vi "Interpolate Real.vi"(0 "Bc":dbl=330.0 format="%_4g", 1 "y":dbl=175.0 format="%_4g", 2 "Mag":dbl=50.0 format="%_4g", 3 "theta":ext=1.950013999999992 format="%_4g", 4 "Initial":dbl[](array[numeric])=[535.0, 450.0] format="%_3g", 5 "g0":dbl=0.30979 format="%_3g", 8 "width":dbl=0.04216999999999992 format="%_3g") -> (7 "sum":dbl(knob)=1360414.7194911004 scale=0.0..30000.0)   [LabVIEW 2016]
panel:
  in  "Tab Control":T1(tab)=enum."Data+Fit"
  out "Skeleton":cluster{"B+i Vsg":cdb[]}[](array[cluster])=[{"B+i Vsg"=[535.0+0.0i, 184.2548459187753+306.77613669047014i, 165.7451540812247+353.22386330952986i, -76.67944631491423+535.0i]}, {"B+i Vsg"=[450.0+0.0i, 184.2548459187753+306.77613669047014i, 165.7451540812247+353.22386330952986i, -13.444317955229593+535.0i]}] {"B+i Vsg" format="%_3g"}
  in  "w":dbl[](array[numeric])=[1.0, 1.0, 1.0]
  out "B":dbl=-0.0009832390037923806 format="%_3g"
  out "gcalc":dbl=1.4433966272486396
  out "XY Graph":cluster{dbl[], dbl[]}[](graph)=[{[0.0, 306.77613669047014, 353.22386330952986, 535.0], [535.0, 184.2548459187753, 165.7451540812247, -76.67944631491423]}, {[0.0, 306.77613669047014, 353.22386330952986, 535.0], [450.0, 184.2548459187753, 165.7451540812247, -13.444317955229593]}]
  in  "i final":dbl=535.0
  in  "i initial":dbl
  in  "Bscale":dbl=-1.0
  out "Data - Fit":dbl[][](graph)
  in  "Mask?":bool=TRUE
  out "Fit":dbl[][](graph)
  in  "Data":dbl[][](graph)=array535x467[249845 elements]
  out "Data - Fit Crop":dbl[][](graph)
  in  "Ny":i32=467
  in  "y0":i32
  in  "Nx":i32=535
  in  "x0":i32
  in  "Mask":dbl[][](graph)=array535x467[249845 elements]
  out "Re Out":dbl[](array[numeric])=[-0.05, 0.05, 0.3]
  out "Out":cdb[](array[numeric])=[-0.05+0.0i, 0.05+0.0i, 0.3+0.0i]
  out "size(s) 2":i32[](array[numeric])=[535, 467]
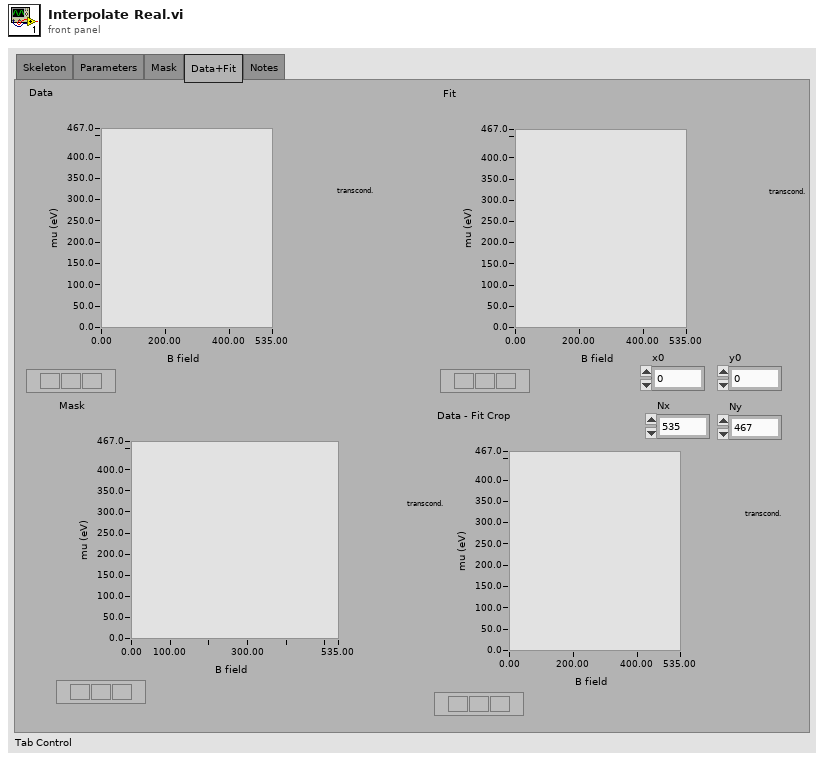
[diagram p1: front panel]
types:
  T1 = enum32{"Skeleton", "Parameters", "Mask", "Data+Fit", "Notes"}
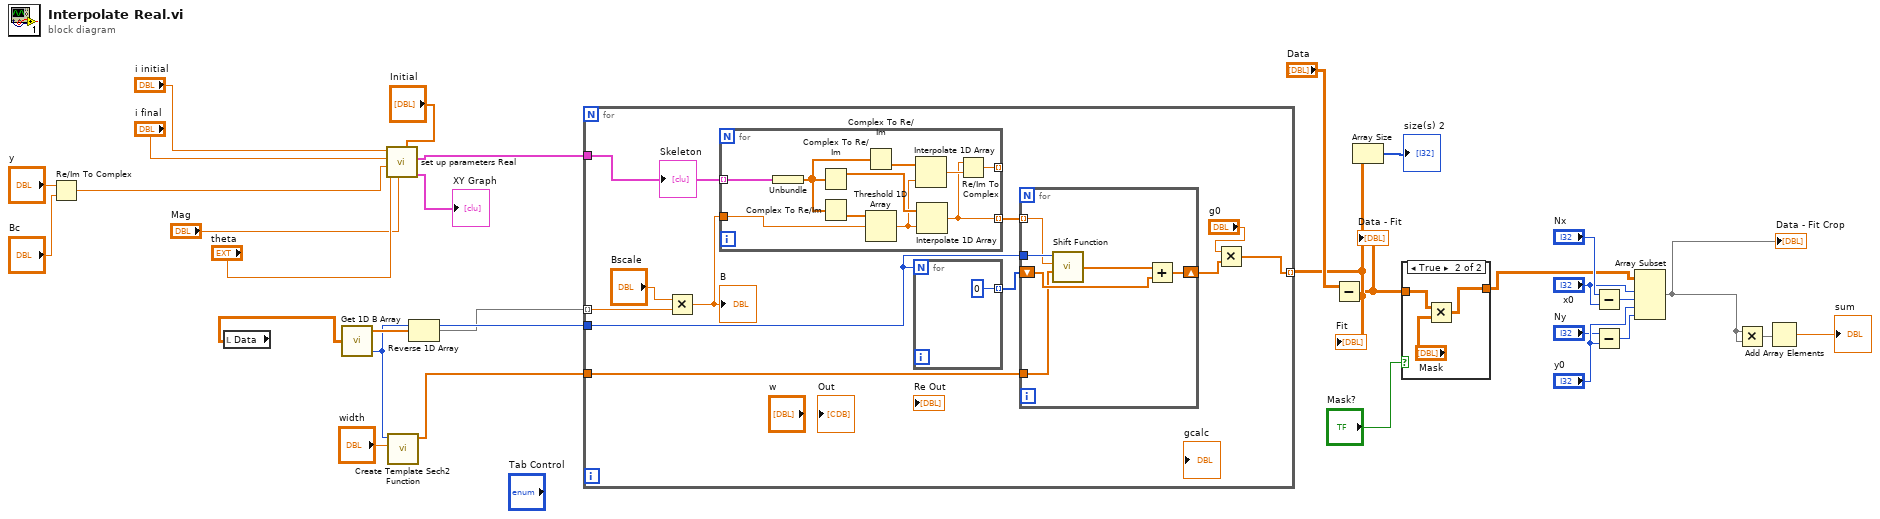
[diagram p0: block diagram]
diagram:
  n1 = Re/Im To Complex(1:"Bc", 2:"y") -> (0:w14:cdb)
  n2 = local read "Data"() -> (w1:dbl[][])
  n3 = call "Get 1D B Array.vi"("B"=w1) -> ("B 1D"=w26:dbl[], "Ny"=w25:i32)  [unwired: 1 out]
  n4 = call "set up parameters Real.vi"("i initial"="i initial", "i final"="i final", "X-point"=w14, "theta"="theta", "Mag"="Mag", "Initial"="Initial") -> ("Skeleton"=w17:cluster{"B+i Vsg":cdb[]}[], "XY Graph"=→"XY Graph":cluster{dbl[], dbl[]}[])  [unwired: 3 in]
  n5 = call "Create Template Sech2 Function.vi"("w"="width", "N"=w25) -> ("Array"=w31:dbl[])  [unwired: 9 in]
  n6 = Reverse 1D Array(array=w26) -> (reversed array=w24:dbl[])
  n7 = for {
    tunnel: [w33] -> w27 mode=indexing
    tunnel: w31 -> [w42]
    tunnel: w25 -> [w37]
    tunnel: w24 -> [w36] mode=indexing
    tunnel: w17 -> [w32]
    n8 = Multiply(x="Bscale", y=w36) -> (x*y=w40:dbl)
    "B" <- w40
    n9 = for {
      tunnel: w32 -> [w59] mode=indexing
      tunnel: w40 -> [w57]
      tunnel: [w51] -> _ mode=indexing
      tunnel: [w50] -> w39 mode=indexing
      n10 = Unbundle(w59) -> ("B+i Vsg"=w56:cdb[])
      n11 = Complex To Re/Im(x + iy=w56) -> (x=w55:dbl[])  [unwired: 1 out]
      n12 = Complex To Re/Im(x + iy=w56) -> (y=w58:dbl[])  [unwired: 1 out]
      n13 = Complex To Re/Im(x + iy=w56) -> (y=w54:dbl[])  [unwired: 1 out]
      n14 = Threshold 1D Array(2:w57, 3:w58) -> (0:w53:dbl)  [unwired: 1 in]
      n15 = Interpolate 1D Array(1:w53, 2:w54) -> (0:w52:dbl)
      n16 = Interpolate 1D Array(1:w53, 2:w55) -> (0:w50:dbl)
      n17 = Re/Im To Complex(1:w52, 2:w50) -> (0:w51:cdb)
    }
    n18 = for {
      N: w37 -> [_]
      tunnel: [0] -> w38 mode=indexing
    }
    n19 = for {
      tunnel: w37 -> [w49]
      tunnel: w39 -> [w48] mode=indexing
      shift-right: [w45] -> w35
      shift-left: w38 -> [w46]
      tunnel: w42 -> [w44]
      n20 = call "Shift Function.vi"("N"=w49, "Vshift"=w48, "Template"=w44) -> ("Waveform Graph"=w47:dbl[])  [unwired: 2 in]
      n21 = Add(x=w47, y=w46) -> (x+y=w45:dbl[])
    }
    n22 = Multiply(x="g0", y=w35) -> (x*y=w33:dbl[])
    "Skeleton" <- w32
  }
  "Fit" <- w27
  n23 = Subtract(x="Data", y=w27) -> (x-y=w15:dbl[][])
  "Data - Fit" <- w15
  n24 = Array Size(array=w27) -> (size(s)=→"size(s) 2":i32[])
  n25 = case shown="True" "Mask?" {
    tunnel: w15 -> [w60 w63]
    tunnel: [w60 w61] -> w3
    frame False {
    }
    frame True {
      n26 = Multiply(x=w63, y="Mask") -> (x*y=w61:dbl[][])
    }
  }
  n27 = Subtract(x="Nx", y="x0") -> (x-y=w8:i32)
  n28 = Subtract(x="Ny", y="y0") -> (x-y=w5:i32)
  n29 = Array Subset(array=w3, index (row)="x0", length (row)=w8, index (col)="y0", length (col)=w5) -> (w2:dbl[][])
  "Data - Fit Crop" <- w2
  n30 = Multiply(x=w2, y=w2) -> (x*y=w16:dbl[][])
  n31 = Add Array Elements(numeric array=w16) -> (sum=→"sum":dbl)
